vi "Transconductance state machine.vi"() -> ()   [LabVIEW 2016] (continued)
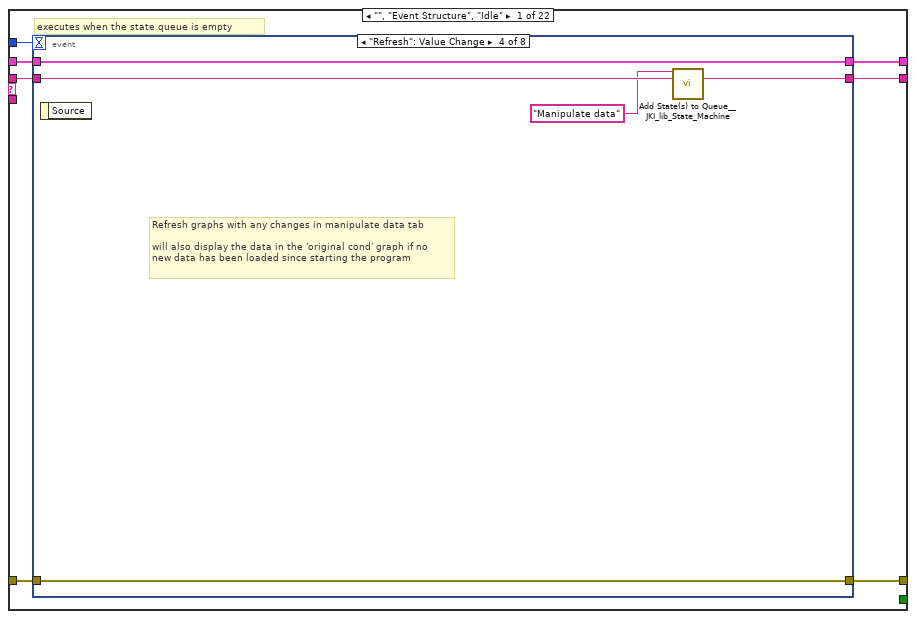
[diagram p2: hidden frame]
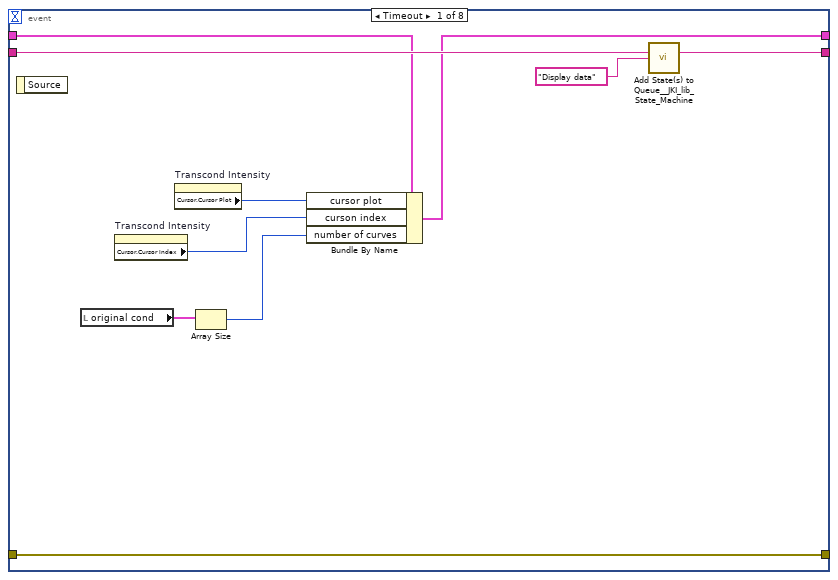
[diagram p3: hidden frame]
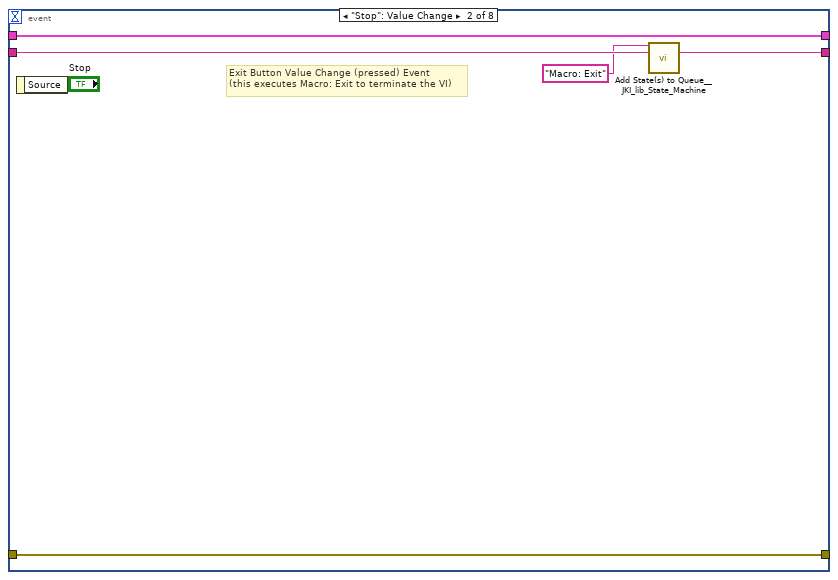
[diagram p4: hidden frame]
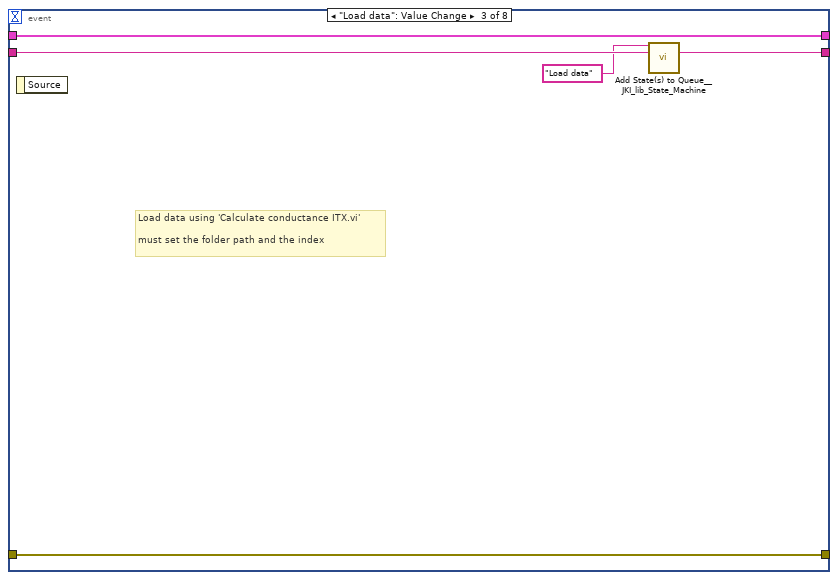
[diagram p5: hidden frame]
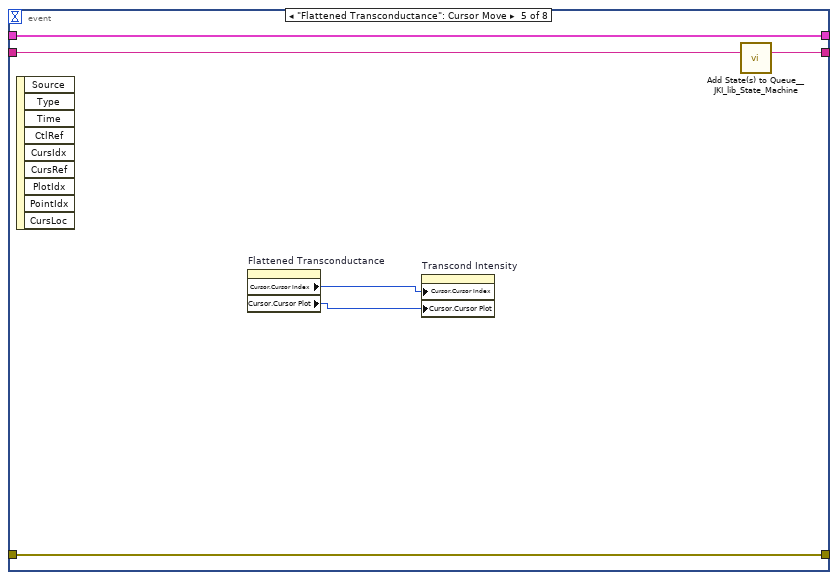
[diagram p6: hidden frame]
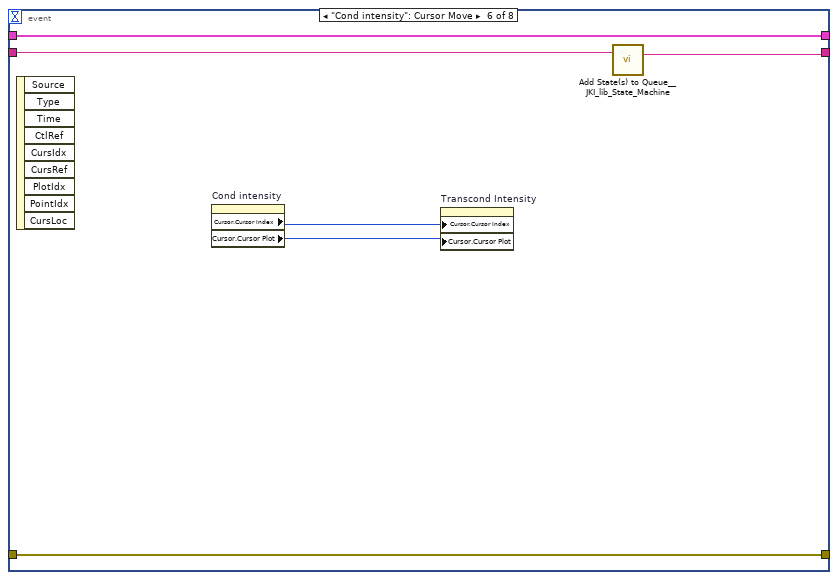
[diagram p7: hidden frame]
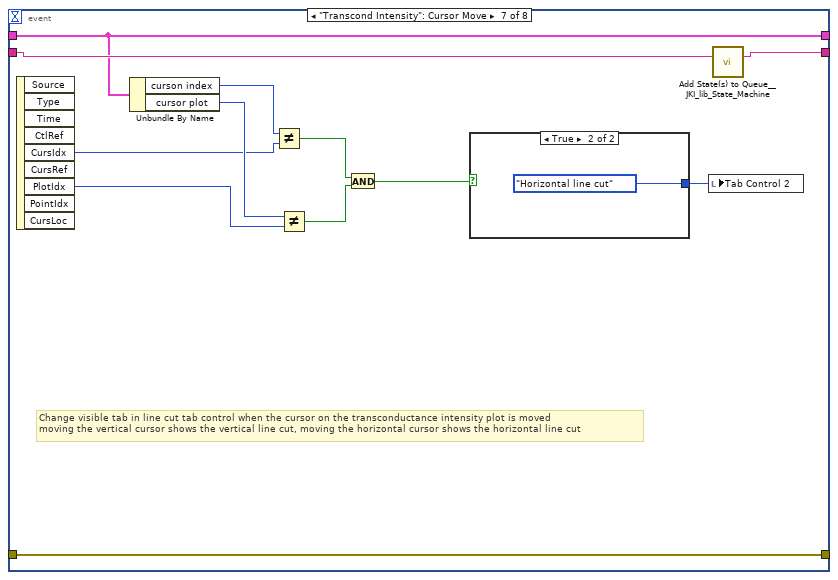
[diagram p8: hidden frame]
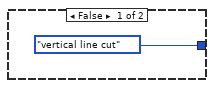
[diagram p9: hidden frame]
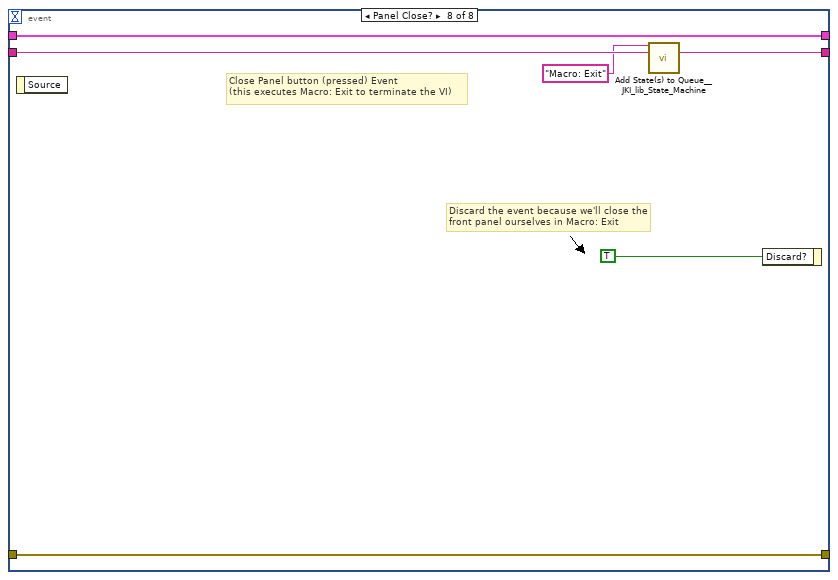
[diagram p10: hidden frame]
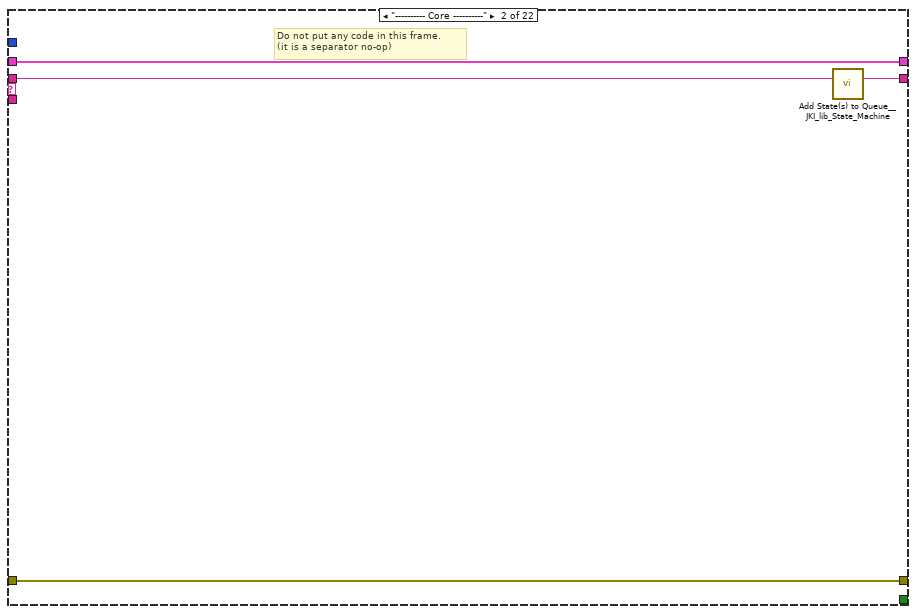
[diagram p11: hidden frame]
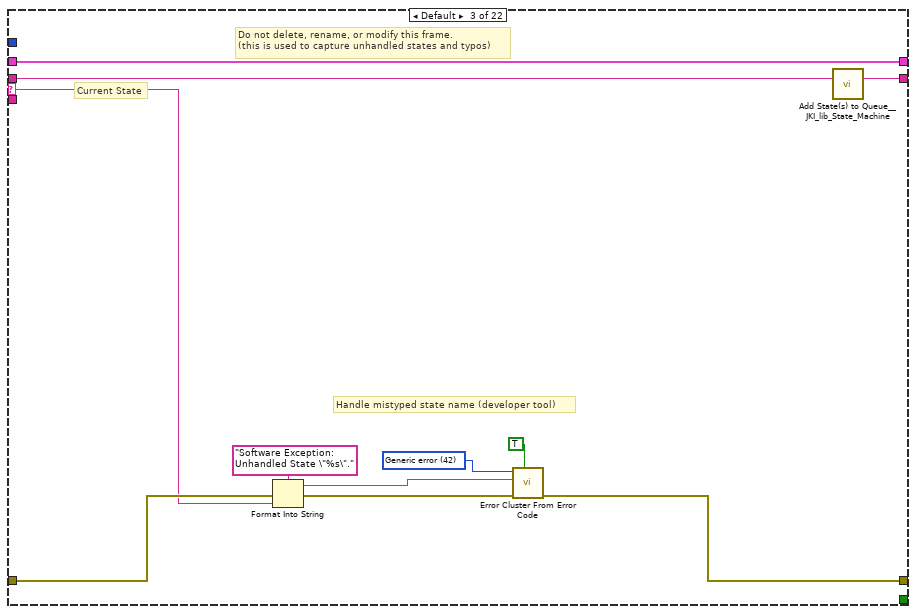
[diagram p12: hidden frame]
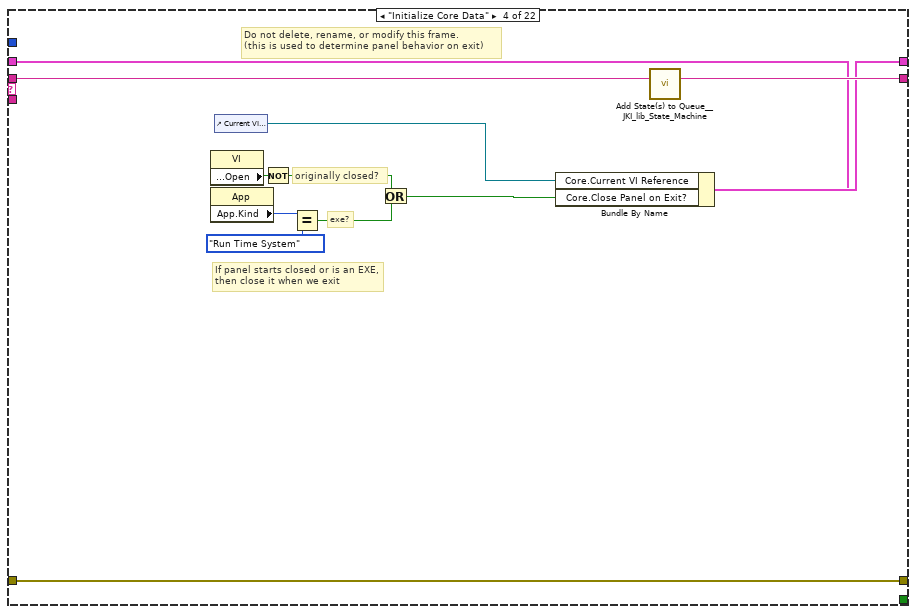
[diagram p13: hidden frame]
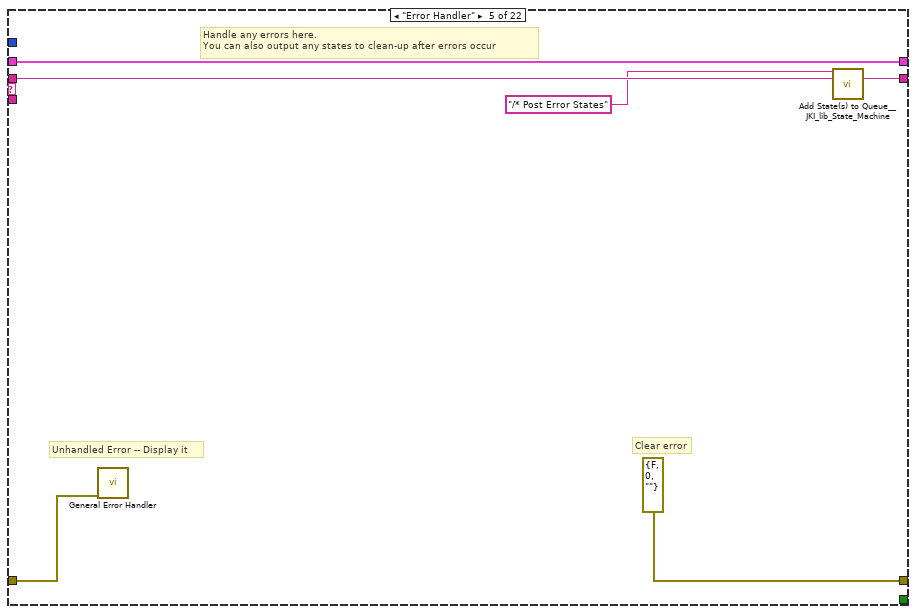
[diagram p14: hidden frame]
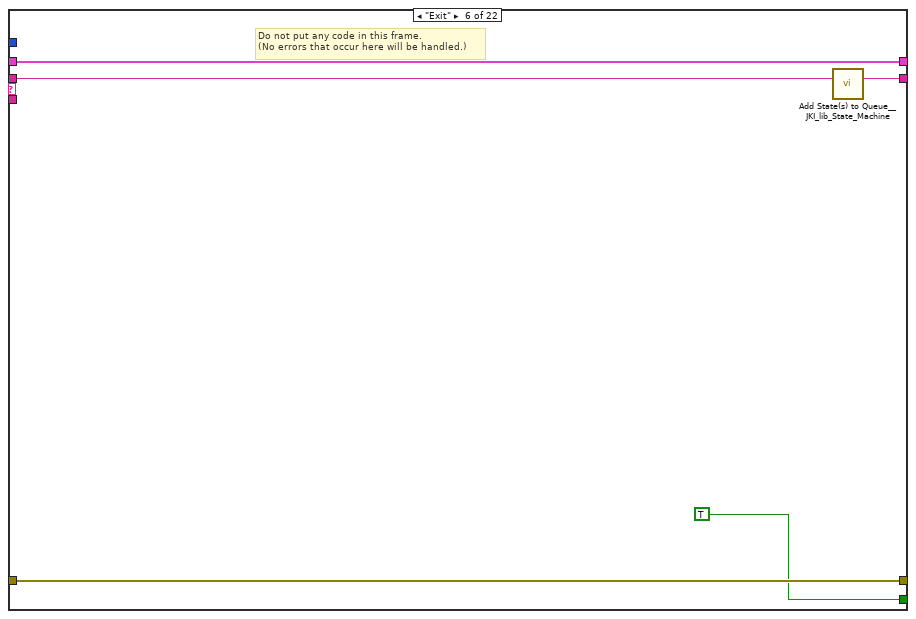
[diagram p15: hidden frame]
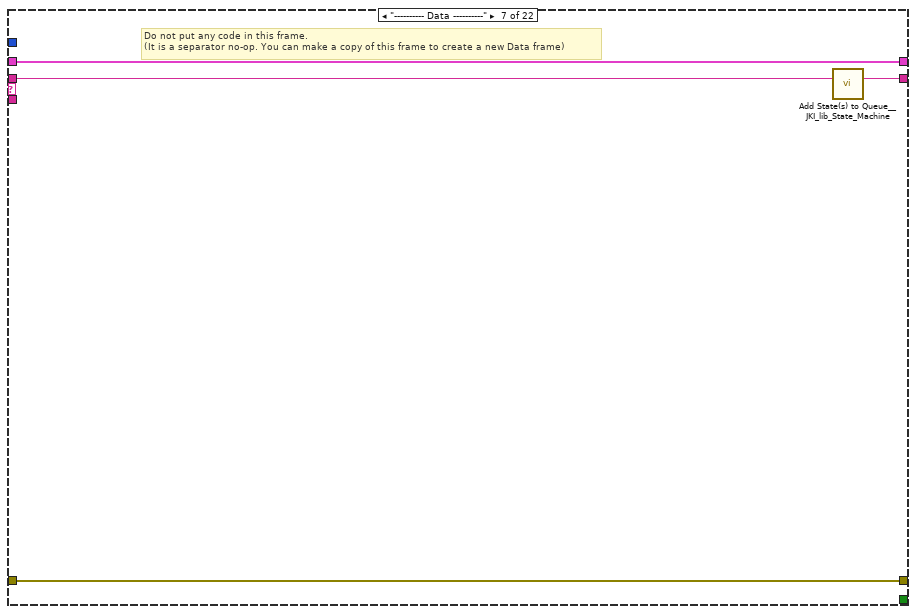
[diagram p16: hidden frame]
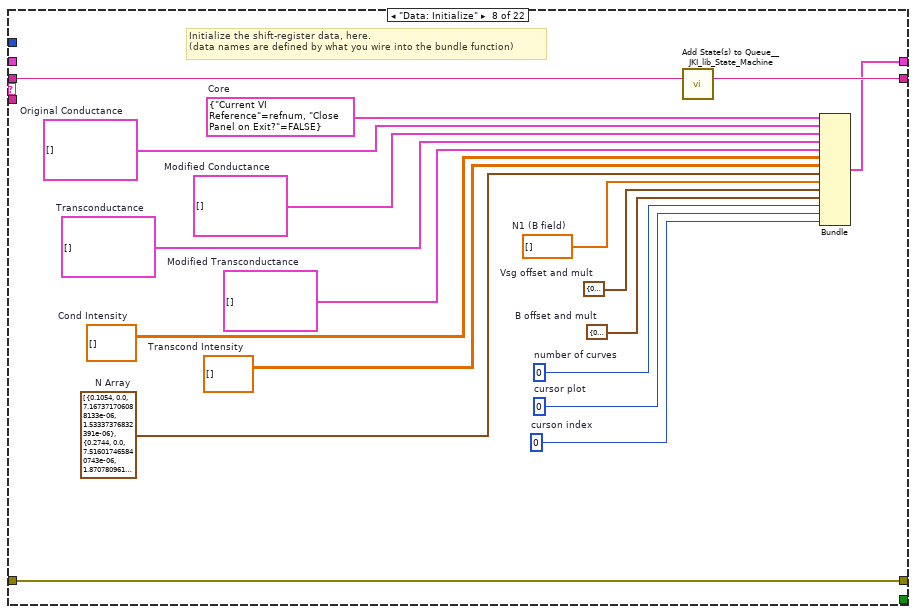
[diagram p17: hidden frame]
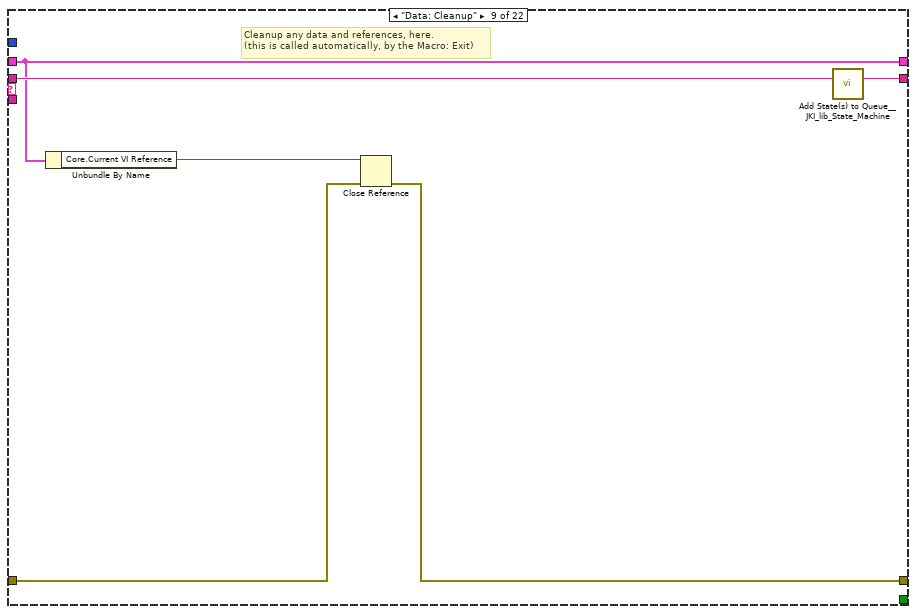
[diagram p18: hidden frame]
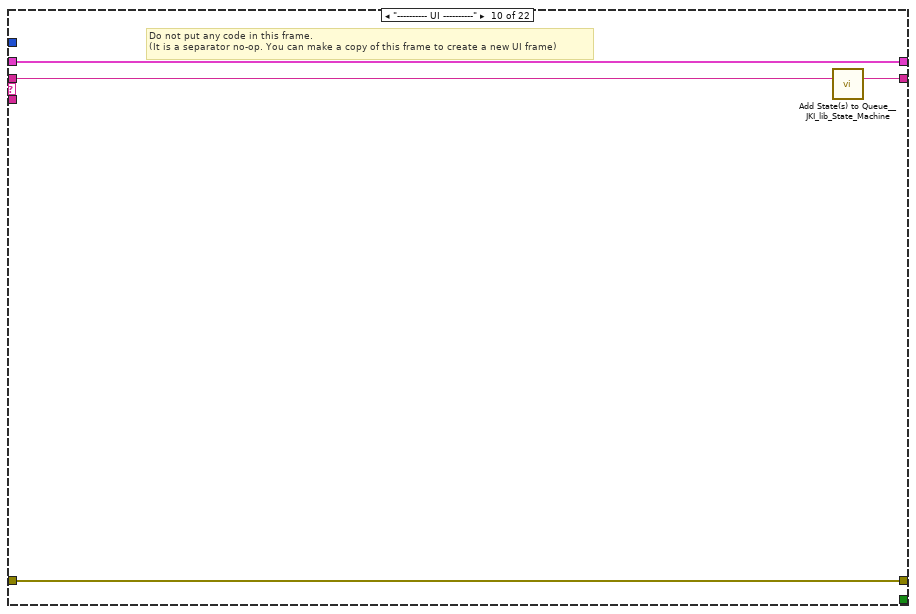
[diagram p19: hidden frame]
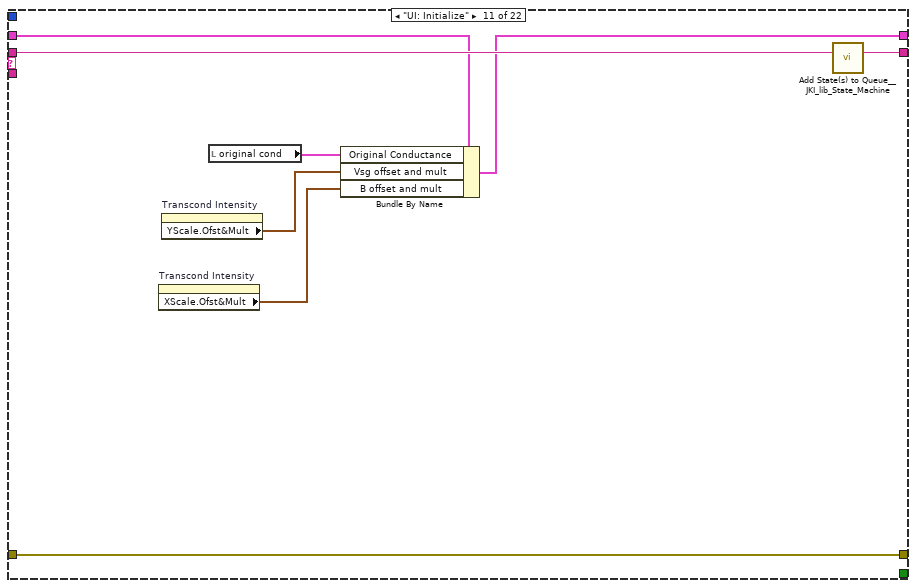
[diagram p20: hidden frame]
          }
        }
        n68 = call <vilib>:"Add State(s) to Queue__JKI_lib_State_Machine.vi"("State(s) in (\"\")"=w161) -> ("States Out"=w160:string)  [unwired: 14 in]
      }
      frame "UI: Front Panel State" {
        # "Argument"
        # "Set Front Panel Open or Closed\n(Usage: \"UI: Front Panel State >> Open|Close\")"
        n69 = Unbundle By Name(w168) -> ("Core.Current VI Reference"=w167:refnum<vi>)
        n70 = case shown="\"Open\", Default" w166 {
          tunnel: w170 -> [w176 w189]
          tunnel: [w178 w190] -> w169
          tunnel: w167 -> [w177 w187]
          frame "Open", Default {
            n71 = property class="VI"(reference=w177, error in=w176) -> (reference out=w174:refnum<vi>, error out=w175:errorcluster, "Front Panel.Open"=w173:bool)
            n72 = case shown="False" w173 {
              tunnel: [w181 w184] -> w178
              tunnel: w175 -> [w180 w184]
              tunnel: w174 -> [w179 _]
              frame False {
                n73 = invoke class="VI" method="FP.Open"(reference=w179, error in=w180, "Activate"=TRUE, "State"=T6."Standard") -> (error out=w181:errorcluster)  [unwired: 1 in, 4 out]
              }
              frame True {
              }
            }
          }
          frame "Close" {
            n74 = property class="VI"(reference=w187, error in=w189) -> (reference out=w186:refnum<vi>, error out=w188:errorcluster, "Front Panel.Open"=w185:bool)
            n75 = case shown="True" w185 {
              tunnel: [w191 w194] -> w190
              tunnel: w188 -> [w191 w193]
              tunnel: w186 -> [_ w192]
              frame False {
              }
              frame True {
                n76 = invoke class="VI" method="FP.Close"(reference=w192, error in=w193) -> (error out=w194:errorcluster)  [unwired: 1 in, 2 out]
              }
            }
          }
        }
        n77 = call <vilib>:"Add State(s) to Queue__JKI_lib_State_Machine.vi"("State(s) in (\"\")"=w172) -> ("States Out"=w171:string)  [unwired: 14 in]
      }
      frame "---------- Macro ----------" {
        # "Do not put any code in this frame.\n(It is a separator no-op. You can make a copy of this frame to create a new Macro frame)"
        n78 = call <vilib>:"Add State(s) to Queue__JKI_lib_State_Machine.vi"("State(s) in (\"\")"=w198) -> ("States Out"=w197:string)  [unwired: 14 in]
      }
      frame "Macro: Initialize" {
        w199 = "Data: Initialize\nInitialize Core Data\nUI: Initialize\nUI: Front Panel State >> Open"  # Data: Initialize Initialize Core Data UI: Initialize UI: Front Panel State >> Open
        # "Initialization Macro\n(This is called once, when the VI starts)"
        n79 = call <vilib>:"Add State(s) to Queue__JKI_lib_State_Machine.vi"("State(s) in Front (\"\")"=w199, "State(s) in (\"\")"=w203) -> ("States Out"=w202:string)  [unwired: 13 in]
      }
      frame "Macro: Exit" {
        # "Exit Macro\n(This is called once, when the VI exits)"
        n80 = Unbundle By Name(w210) -> ("Core.Close Panel on Exit?"=w209:bool)
        n81 = Select(t="UI: Front Panel State >> Close", s=w209, f="") -> (s? t:f=w206:string)
        n82 = call <vilib>:"Add State(s) to Queue__JKI_lib_State_Machine.vi"("State(s) in (\"\")"=w206, "State(s) at Back (\"\")"="Data: Cleanup\nExit") -> ("States Out"=w204:string)  [unwired: 13 in]
        n83 = call <vilib>:"Add State(s) to Queue__JKI_lib_State_Machine.vi"("State(s) in Front (\"\")"=w204, "State(s) in (\"\")"=w213) -> ("States Out"=w212:string)  [unwired: 13 in]
      }
      frame "---------- New Category ----------" {
        # "Template Separator\n(You can make a copy of, or modify, this frame)"
        n84 = call <vilib>:"Add State(s) to Queue__JKI_lib_State_Machine.vi"("State(s) in (\"\")"=w217) -> ("States Out"=w216:string)  [unwired: 14 in]
      }
      frame "Load data" {
        # "Load conductance data"
        # "calculate B offset and multiplier\nfor intensity plots"
        # "calculate Vsg offset and multiplier for intensity plots"
        n85 = local read "File or Folder Path"() -> (w253:path)
        n86 = local read "index"() -> (w252:T3)
        n87 = call "Calculate conductance ITX.vi"("progress bar?"=TRUE, "length"="length", "offset"="offset", "index"=w252, "File or Folder Path"=w253) -> ("N Array"=w220:T9, "Comments"=→"Comments":string, "A vs D"=w224:cluster{dbl[], dbl[]}[])  [unwired: 1 in, 3 out]
        n88 = Index Array(array=w224) -> (element=w244:cluster{dbl[], dbl[]})  [unwired: 1 in]
        n89 = for {
          tunnel: w220 -> [w258] mode=indexing
          tunnel: [w257] -> w240 mode=indexing
          n90 = Unbundle By Name(w258) -> ("N1"=w257:dbl)
        }
        n91 = Array Size(array=w224) -> (size(s)=w229:i32)
        n92 = Unbundle(w244) -> (w247:dbl[])  [unwired: 1 out]
        n93 = local write "original cond"(w224) -> ()
        n94 = Array Size(array=w240) -> (size(s)=w239:i32)
        n95 = Index Array(array=w247, index #1=1 ("index"), index #2=0 ("index")) -> (element #1=w246:dbl, element #2=w245:dbl)
        n96 = Array Max & Min(array=w247) -> (min value=w243:dbl)  [unwired: 3 out]
        n97 = Decrement(x=w239) -> (x-1=w238:i32)
        n98 = Subtract(x=w246, y=w245) -> (x-y=w242:dbl)
        n99 = Index Array(array=w240, index #1=0 ("index"), index #2=w238) -> (element #1=w232:dbl, element #2=w233:dbl)
        n100 = Bundle(w243, w242) -> (w241:cluster{dbl, dbl})  [unwired: 1 in]
        n101 = Subtract(x=w232, y=w233) -> (x-y=w231:dbl)
        n102 = Less?(x=w232, y=w233) -> (x < y?=w236:bool)
        n103 = Absolute Value(x=w231) -> (abs(x)=w230:dbl)
        n104 = Select(t=1.0, s=w236, f=-1.0) -> (s? t:f=w227:dbl)
        n105 = Divide(x=w230, y=w229) -> (x/y=w228:dbl)
        n106 = Multiply(x=w227, y=w228) -> (x*y=w226:dbl)
        n107 = Bundle("N1"=w232, w226) -> (w225:cluster{"N1":dbl, dbl})  [unwired: 1 in]
        n108 = Bundle By Name(cluster=w223, "Vsg offset and mult"=w241, "number of curves"=w229, "Original Conductance"=w224, "N Array"=w220, "N1 (B field)"=w240, "B offset and mult"=w225) -> (w251:T8)
        n109 = call <vilib>:"Add State(s) to Queue__JKI_lib_State_Machine.vi"("State(s) in (\"\")"=w256, "State(s) at Back (\"\")"="Manipulate data" ("State(s) at Back (\"\")")) -> ("States Out"=w255:string)  [unwired: 13 in]
      }
      frame "Manipulate data" {
        n110 = Unbundle By Name(w261) -> ("Original Conductance"=w265:T4)
        n111 = case shown="True" "restrict range?" {
          tunnel: w265 -> [w280 w282]
          tunnel: [w280 w281] -> w262
          frame False {
          }
          frame True {
            # "restrict the range of the data"
            n112 = for {
              tunnel: w282 -> [w290] mode=indexing
              tunnel: [w283] -> w281 mode=indexing
              w287 = u16 0 items=["Y", "X", "X and Y"] ("range type")
              n113 = Unbundle(w290) -> ("Vfast"=w289:dbl[], "Decimated Array"=w288:dbl[])
              n114 = call-poly <vilib>:"Remove Outliers.vi"("Y"=w288, "X"=w289, "range type"=w287, "Range"="conductance range") -> ("Y Out"=w285:dbl[], "X Out"=w284:dbl[])  [unwired: 7 in, 3 out]
              n115 = Bundle("X Out"=w284, "Y Out"=w285) -> (w283:cluster{"X Out":dbl[], "Y Out":dbl[]})  [unwired: 1 in]
            }
          }
        }
        n116 = case shown="True" "Filter?" {
          tunnel: w262 -> [w270 w272]
          tunnel: [w270 w271] -> w260
          frame False {
          }
          frame True {
            # "option to filter the conductance data"
            n117 = for {
              tunnel: w272 -> [w279] mode=indexing
              tunnel: [w275] -> w271 mode=indexing
              n118 = Unbundle(w279) -> ("X Out"=w276:dbl[], "Y Out"=w278:dbl[])
              n119 = call-poly <vilib>:"Chebyshev Filter.vi"("filter type"=Filter_Passband_Type."Lowpass", "low cutoff freq: fl"="low cutoff freq: fh 2", "X"=w278) -> ("Filtered X"=w277:dbl[])  [unwired: 7 in, 1 out]
              n120 = Bundle("X Out"=w276, "Filtered X"=w277) -> (w275:cluster{"X Out":dbl[], "Filtered X":dbl[]})  [unwired: 1 in]
            }
          }
        }
        n121 = Bundle By Name(cluster=w261, "Modified Conductance"=w260) -> (w259:T8)
        n122 = call <vilib>:"Add State(s) to Queue__JKI_lib_State_Machine.vi"("State(s) in (\"\")"=w269, "State(s) at Back (\"\")"="Transconductance" ("State(s) at Back (\"\")")) -> ("States Out"=w268:string)  [unwired: 13 in]
      }
      frame "Transconductance" {
        n123 = Unbundle By Name(w294) -> ("Modified Conductance"=w295:T4)
        n124 = for {
          tunnel: w295 -> [w300] mode=indexing
          tunnel: [w299] -> w293 mode=indexing
          n125 = call <userlib>:"differential.vi"("Numeric"="derivative points", "dy/dx vs x"="dy/dx vs x", "A vs B 2"=w300) -> ("A vs B 3"=w299:T12)  [unwired: 1 in]
        }
        n126 = Bundle By Name(cluster=w294, "Transconductance"=w293) -> (w292:T8)
        n127 = call <vilib>:"Add State(s) to Queue__JKI_lib_State_Machine.vi"("State(s) in (\"\")"=w298, "State(s) at Back (\"\")"="Flatten Transconductance" ("State(s) at Back (\"\")")) -> ("States Out"=w297:string)  [unwired: 13 in]
      }
      frame "Flatten Transconductance" {
        n128 = Unbundle By Name(w313) -> ("Transconductance"=w308:T4, "Vsg offset and mult"=w311:cluster{dbl, dbl}, "number of curves"=w307:i32)
        "number of curves" <- w307
        n129 = Initialize Array(0.0 ("element"), w307) -> (w305:dbl[])
        n130 = Add(x=w305, y="manual offset array") -> (x+y=w303:dbl[])
        n131 = for {
          tunnel: w308 -> [w334] mode=indexing
          tunnel: w311 -> [w324]
          tunnel: [w321] -> w310 mode=indexing
          tunnel: w303 -> [w318] mode=indexing
          n132 = Unbundle(w324) -> (w322:dbl)  [unwired: 1 out]
          n133 = Unbundle(w334) -> ("Vfast"=w329:dbl[], "Decimated Array"=w327:dbl[])
          n134 = call <vilib>:"Peak Detector.vi"("peaks/valleys"=enum32{"Peaks", "Valleys"}."Peaks", "width"="width", "threshold"="threshold", "X"=w327) -> ("Locations"=w331:dbl[])  [unwired: 3 in, 4 out]
          n135 = Index Array(array=w331) -> (element=w330:dbl)  [unwired: 1 in]
          n136 = Index Array(array=w329, index=w330) -> (element=w328:dbl)
          n137 = Subtract(x=w329, y=w328) -> (x-y=w319:dbl[])
          n138 = Add(x=w319, y=w318) -> (x+y=w317:dbl[])
          n139 = Bundle(w317, "Decimated Array"=w327) -> (w323:cluster{dbl[], "Decimated Array":dbl[]})  [unwired: 1 in]
          n140 = call <userlib>:"Decimate_VS_X_Value.vi"("XY Graph kind 1"=w323, "X Step"=w322, "X High"="X High", "X Low"="X Low") -> ("Interpreted"=w321:cluster{dbl[], dbl[]})  [unwired: 6 in, 1 out]
        }
        n141 = Bundle By Name(cluster=w313, "Modified Transconductance"=w310) -> (w312:T8)
        n142 = call <vilib>:"Add State(s) to Queue__JKI_lib_State_Machine.vi"("State(s) in (\"\")"=w316, "State(s) at Back (\"\")"="Display data" ("State(s) at Back (\"\")")) -> ("States Out"=w315:string)  [unwired: 13 in]
      }
      frame "Display data" {
        n143 = Unbundle By Name(w354) -> ("Modified Conductance"=w346:T4, "Transconductance"=w352:T4, "Modified Transconductance"=w350:T4, "Vsg offset and mult"=w336:cluster{dbl, dbl}, "B offset and mult"=w337:cluster{dbl, dbl}, "N1 (B field)"=w335:dbl[])
        "modified transconductance" <- w350
        n144 = property on="Flattened Transconductance" class="IntGraph (strict)"("XScale.Ofst&Mult"=w337) -> ()  [unwired: 2 in, 2 out]
        n145 = property on="Flattened Transconductance" class="IntGraph (strict)"("YScale.Ofst&Mult"=w336) -> ()  [unwired: 2 in, 2 out]
        n146 = property on="Cond intensity" class="IntGraph (strict)"("XScale.Ofst&Mult"=w337) -> ()  [unwired: 2 in, 2 out]
        n147 = property on="Transcond Intensity" class="IntGraph (strict)"("YScale.Ofst&Mult"=w336) -> ()  [unwired: 2 in, 2 out]
        n148 = property on="Transcond Intensity" class="IntGraph (strict)"("XScale.Ofst&Mult"=w337) -> ()  [unwired: 2 in, 2 out]
        n149 = property on="Cond intensity" class="IntGraph (strict)"("YScale.Ofst&Mult"=w336) -> ()  [unwired: 2 in, 2 out]
        n150 = for {
          tunnel: w346 -> [w377] mode=indexing
          tunnel: w352 -> [w376] mode=indexing
          tunnel: [w371] -> w353 mode=indexing
          tunnel: [w364] -> w340 mode=indexing
          tunnel: [w370] -> w349 mode=indexing
          tunnel: [w367] -> w351 mode=indexing
          tunnel: w350 -> [w366] mode=indexing
          tunnel: [w365] -> w345 mode=indexing
          i -> [w361]
          n151 = Unbundle(w366) -> ("Decimated Array"=w365:dbl[])  [unwired: 1 out]
          n152 = Unbundle(w377) -> ("Vfast"=w374:dbl[], "Decimated Array"=w371:dbl[])
          n153 = Unbundle(w376) -> ("Vfast"=w363:dbl[], "Decimated Array"=w364:dbl[])
          n154 = Multiply(x="offset cond (horizontal)", y=w361) -> (x*y=w373:dbl)
          n155 = Multiply(x="offset trans (vertical)", y=w361) -> (x*y=w368:dbl)
          n156 = Add(x=w374, y=w373) -> (x+y=w372:dbl[])
          n157 = Add(x=w364, y=w368) -> (x+y=w362:dbl[])
          n158 = Bundle(w372, "Decimated Array"=w371) -> (w370:cluster{dbl[], "Decimated Array":dbl[]})  [unwired: 1 in]
          n159 = Bundle("Vfast"=w363, w362) -> (w367:cluster{"Vfast":dbl[], dbl[]})  [unwired: 1 in]
        }
        "Cond intensity" <- w353
        "Transcond Intensity" <- w340
        "Flattened Transconductance" <- w345
        n160 = property on="Transcond Intensity" class="IntGraph (strict)"() -> ("Cursor.Cursor Y"=→"Vsg (V)":dbl)  [unwired: 2 in, 2 out]
        n161 = property on="Transcond Intensity" class="IntGraph (strict)"() -> ("Cursor.Cursor X"=→"B field (T)":dbl)  [unwired: 2 in, 2 out]
        n162 = property on="Transcond Intensity" class="IntGraph (strict)"() -> ("Cursor.Cursor Plot"=w341:i32)  [unwired: 2 in, 2 out]
        n163 = property on="Transcond Intensity" class="IntGraph (strict)"() -> ("Cursor.Cursor Index"=w347:i32)  [unwired: 2 in, 2 out]
        n164 = local write "Transconductance"(w351) -> ()
        n165 = Transpose 2D Array(2D array=w340) -> (transposed array=w344:dbl[][])
        n166 = local write "Conductance"(w349) -> ()
        n167 = Index Array(array=w346, index=w347) -> (element=→"Conductance curve\nvertical line cut":cluster{"Vfast":dbl[], "Decimated Array":dbl[]})
        n168 = for {
          tunnel: w344 -> [w359] mode=indexing
          tunnel: w335 -> [w360]
          tunnel: [w358] -> w343 mode=indexing
          n169 = Bundle("N1 (B field)"=w360, w359) -> (w358:cluster{"N1 (B field)":dbl[], dbl[]})  [unwired: 1 in]
        }
        n170 = Index Array(array=w343, index=w341) -> (element=→"Transcond curve\nhorizontal line cut":cluster{"N1 (B field)":dbl[], dbl[]})
        n171 = call <vilib>:"Add State(s) to Queue__JKI_lib_State_Machine.vi"("State(s) in (\"\")"=w357) -> ("States Out"=w356:string)  [unwired: 14 in]
      }
    }
  }
